vi "UHR-Fleezers Control (host) - 12.8.1.vi"() -> ()   [LabVIEW 2012] (continued)
        n1295 = Path To String(path=w1922) -> (string=w1921:string)
        n1296 = Concatenate Strings(w1921, "\\current.cal" ("string")) -> (w1919:string)
        n1297 = String To Path(string=w1919) -> (path=w1918:path)
        n1298 = Open/Create/Replace File(file path (use dialog)=w1918, operation (0:open)=T33."open", access (0:read/write)=enum16{"read/write", "read-only", "write-only"}."read-only") -> (refnum out=w1926:refnum<file>, error out=w1912:errorcluster)  [unwired: 1 in, 3 out]
        n1299 = Deny Access(4:w1912, 7:w1926) -> (0:w1911:errorcluster, 3:w1917:refnum<file>)  [unwired: 1 out]
        n1300 = Read from Binary File(5:0.0, 8:w1911, 9:T32."big-endian, network order" ("byte order (0:big-endian, network order)"), 10:-1 ("count (1)"), 11:w1917) -> (0:w1910:errorcluster, 2:w1908:dbl[], 3:w1913:refnum<file>)  [unwired: 2 out]
        n1301 = Array To Cluster(array=w1908) -> (cluster=w1907:T35)
        n1302 = Unbundle(w1907) -> ("[0]"=w1901:dbl, "[1]"=w1895:dbl, "[2]"=w1899:dbl, "[3]"=w1893:dbl, "[4]"=w1906:dbl, "[5]"=w1905:dbl)
        n1303 = Close File(refnum=w1913, error in=w1910) -> (error out=→"Read cal error":errorcluster)  [unwired: 1 out]
        n1304 = Multiply(x=w1906, y=w1904) -> (x*y=w1900:dbl)
        n1305 = Multiply(x=w1905, y=w1904) -> (x*y=w1894:dbl)
        n1306 = Bundle By Name(cluster="T1 calibration", "T1 alpha_x (nm/V)"=w1901, "T1 offset_x (mV)"=w1900, "T1 kappa_x (pN/nm)"=w1899) -> (w1898:T6)
        n1307 = Bundle By Name(cluster="T2 calibration", "T2 alpha_x (nm/V)"=w1895, "T2 offset_x (mV)"=w1894, "T2 kappa_x (pN/nm)"=w1893) -> (w1896:T5)
        n1308 = local write "T1 calibration"(w1898) -> ()
        n1309 = local write "T2 calibration"(w1896) -> ()
      }
      event "Abort MCL Scan": Value Change {
        n1310 = event-data() -> ()  [unwired: 7 out]
        n1311 = local write "MCL Scanning"(FALSE ("MCL Scanning")) -> ()
        n1312 = xnode "Read/Write Control"("FPGA VI Reference In"=w1927, "Abort scan (MCL)"="Abort MCL Scan") -> ("error out"=w1930:errorcluster)  [unwired: 1 in, 1 out]
      }
      event "Update Count (MCL)": Value Change {
        n1313 = event-data() -> ()  [unwired: 7 out]
        n1314 = xnode "Read/Write Control"("FPGA VI Reference In"=w1931, "MCL count"="Update Count (MCL)") -> ("error out"=w1933:errorcluster)  [unwired: 1 in, 1 out]
      }
      event "+ phase (MCL)", "- phase (MCL)": Value Change {
        n1315 = event-data() -> ()  [unwired: 7 out]
        n1316 = Or(x="- phase (MCL)", y="+ phase (MCL)") -> (x .or. y?=w1937:bool)
        n1317 = Negate(x="Phase adjust (MCL)") -> (-x=w1943:i16)
        n1318 = Select(t=w1943, s="+ phase (MCL)", f="Phase adjust (MCL)") -> (s? t:f=w1941:i16)
        n1319 = xnode "Read/Write Control"("FPGA VI Reference In"=w1934, "Phase count adjustment (MCL)"=w1941) -> ("FPGA VI Reference Out"=w1938:T24, "error out"=w1939:errorcluster)  [unwired: 1 in]
        n1320 = xnode "Read/Write Control"("FPGA VI Reference In"=w1938, "error in"=w1939, "+ phase (MCL)"=w1937) -> ("error out"=w1936:errorcluster)  [unwired: 1 out]
      }
      event "Abort AOD Scan": Value Change {
        n1321 = event-data() -> ()  [unwired: 7 out]
        n1322 = xnode "Read/Write Control"("FPGA VI Reference In"=w1944, "Abort scan"="Abort AOD Scan") -> ("error out"=w1946:errorcluster)  [unwired: 1 in, 1 out]
      }
      event "Continuous AOD Scanning": Value Change {
        n1323 = event-data() -> ()  [unwired: 7 out]
        n1324 = xnode "Read/Write Control"("FPGA VI Reference In"=w1947, "Cont. Scan"="Continuous AOD Scanning") -> ("error out"=w1949:errorcluster)  [unwired: 1 in, 1 out]
      }
      event "Index": Value Change {
        n1325 = event-data() -> ()  [unwired: 7 out]
        n1326 = call "Create new save file.vi"("Insert"="", "Ext"=".dat" ("string"), "Index In"="Index") -> ("Path Out"=→"Save file name":path, "Index Out"=w1950:dbl)
        "Save index" <- w1950
        n1327 = local write "Index"(w1950) -> ()
      }
      event "AO1", "AO2": Value Change {
        w1964 = 10.0 ("y")
        w1963 = 32767.0 ("y")
        n1328 = event-data() -> ()  [unwired: 7 out]
        n1329 = local read "AO2"() -> (w1962:dbl)
        n1330 = local read "AO1"() -> (w1959:dbl)
        n1331 = Multiply(x=w1959, y=w1963) -> (x*y=w1958:dbl)
        n1332 = Multiply(x=w1962, y=w1963) -> (x*y=w1961:dbl)
        n1333 = Divide(x=w1958, y=w1964) -> (x/y=w1957:dbl)
        n1334 = Divide(x=w1961, y=w1964) -> (x/y=w1960:dbl)
        n1335 = To Word Integer(number=w1957) -> (16bit integer=w1965:i16)
        n1336 = To Word Integer(number=w1960) -> (16bit integer=w1966:i16)
        n1337 = xnode "Read/Write Control"("FPGA VI Reference In"=w1955, "AO1"=w1965, "AO2"=w1966) -> ("error out"=w1956:errorcluster)  [unwired: 1 in, 1 out]
      }
      event "Inject Pump 1": Value Change {
        n1338 = event-data() -> ()  [unwired: 7 out]
        n1339 = local read "Use Harvard pumps\nfor beads (else Chemyx)"() -> (w1968:bool)
        n1340 = case shown="True" w1968 {
          tunnel: "Inject Pump 1" -> [w1972 w2010]
          tunnel: w1967 -> [_ w2011]
          frame False {
            n1341 = local read "Pump write delay (ms)"() -> (w1971:dbl)
            n1342 = local read "Chemyx Syringe Pump Serial Port"() -> (w1970:refnum<visa-resource-name>)
            n1343 = case shown="True" w1972 {
              tunnel: w1971 -> [w1978 w1992]
              tunnel: w1970 -> [w1975 w1991]
              frame False {
                n1344 = flat-sequence {
                  tunnel: w1975 -> [w1979]
                  tunnel: [w1979] -> w1976
                  tunnel: w1978 -> [_]
                  tunnel: [w1982] -> w1977
                  tunnel: w1976 -> [w1982]
                  tunnel: w1977 -> [w1983]
                  tunnel: [w1983] -> w1973
                  tunnel: [w1985] -> w1974
                  tunnel: w1973 -> [w1985]
                  tunnel: w1974 -> [w1987]
                  frame #0 {
                    n1345 = call "Write to pump.vi"("string"="enter pump1", "VISA resource name"=w1979) -> ()  [unwired: 1 out]
                  }
                  frame #1 {
                    n1346 = Wait (ms)(milliseconds to wait="Pump pause delay (ms)") -> ()  [unwired: 1 out]
                  }
                  frame #2 {
                    n1347 = call "Write to pump.vi"("string"="stop", "VISA resource name"=w1983) -> ()  [unwired: 1 out]
                  }
                  frame #3 {
                    n1348 = Wait (ms)(milliseconds to wait=u32 500) -> ()  [unwired: 1 out]
                  }
                  frame #4 {
                    n1349 = call "Write to pump.vi"("string"="stop", "VISA resource name"=w1987) -> ()  [unwired: 1 out]
                  }
                }
              }
              frame True {
                n1350 = flat-sequence {
                  tunnel: w1991 -> [w2001]
                  tunnel: w1992 -> [w1996]
                  tunnel: w1992 -> [w2003]
                  tunnel: w1991 -> [w2004]
                  tunnel: [w2004] -> w1989
                  tunnel: [w2006] -> w1990
                  tunnel: w1989 -> [w2006]
                  tunnel: w1990 -> [w2008]
                  frame #0 {
                    n1351 = local read "All Pump Parameters"() -> (w1995:T7)
                    n1352 = Unbundle By Name(w1995) -> ("Pump 1"=w2002:T36)
                    n1353 = call "Set pump parameters.vi"("Pump write delay (ms)"=w1996, "Volume (uL)"="Ch 1 Inject Volume (uL)", "Rate (uL/h)"="Ch 1 Inject Rate (ul/h)", "Units"=4.0, "Pump #"=1.0, "Pump Parameters In"=w2002, "VISA resource name"=w2001) -> ("Pump Parameters Out"=w1994:T36)  [unwired: 3 in]
                    n1354 = Bundle By Name(cluster=w1995, "Pump 1"=w1994) -> (w1993:T7)
                    n1355 = local write "All Pump Parameters"(w1993) -> ()
                  }
                  frame #1 {
                    n1356 = Wait (ms)(milliseconds to wait=w2003) -> ()  [unwired: 1 out]
                  }
                  frame #2 {
                    n1357 = call "Write to pump.vi"("string"="start", "VISA resource name"=w2004) -> ()  [unwired: 1 out]
                  }
                  frame #3 {
                    n1358 = Wait (ms)(milliseconds to wait=u32 500) -> ()  [unwired: 1 out]
                  }
                  frame #4 {
                    n1359 = call "Write to pump.vi"("string"="start", "VISA resource name"=w2008) -> ()  [unwired: 1 out]
                  }
                }
              }
            }
          }
          frame True {
            n1360 = case shown="False" w2010 {
              tunnel: w2011 -> [w2012 w2022]
              frame False {
                n1361 = flat-sequence {
                  tunnel: w2012 -> [w2014]
                  frame #0 {
                    n1362 = local write "Flushing P1"(FALSE ("Flushing P1")) -> ()
                    n1363 = Concatenate Strings("stop" ("string"), "\r") -> (w2016:string)
                    n1364 = VISA Write(VISA resource name=w2014, write buffer=w2016) -> ()  [unwired: 1 in, 3 out]
                  }
                  frame #1 {
                    n1365 = property on="Clear Volume P1" class="Bool (strict)"("Val(Sgnl)"=TRUE ("Value (Signaling)")) -> ()  [unwired: 2 in, 2 out]
                  }
                }
              }
              frame True {
                n1366 = local read "Normal Flow Rate (ul/h) P1"() -> (w2020:dbl)
                n1367 = Number To Decimal String(number=w2020) -> (decimal integer string=w2026:string)  [unwired: 1 in]
                n1368 = Concatenate Strings("irate  " ("string"), w2026, " u/h" ("string"), "\r") -> (w2024:string)
                n1369 = VISA Write(VISA resource name=w2022, write buffer=w2024) -> (VISA resource name out=w2021:refnum<visa-resource-name>)  [unwired: 1 in, 2 out]
                n1370 = Concatenate Strings("irun" ("string"), "\r") -> (w2028:string)
                n1371 = VISA Write(VISA resource name=w2021, write buffer=w2028) -> ()  [unwired: 1 in, 3 out]
              }
            }
          }
        }
      }
      event "Inject Pump 3": Value Change {
        n1372 = event-data() -> ()  [unwired: 7 out]
        n1373 = local read "Use Harvard pumps\nfor beads (else Chemyx)"() -> (w2031:bool)
        n1374 = case shown="True" w2031 {
          tunnel: "Inject Pump 3" -> [w2035 w2074]
          tunnel: w2030 -> [_ w2073]
          frame False {
            n1375 = local read "Pump write delay (ms)"() -> (w2034:dbl)
            n1376 = case shown="True" w2035 {
              tunnel: w2034 -> [w2041 w2055]
              tunnel: "Chemyx Syringe Pump Serial Port" -> [w2038 w2054]
              frame False {
                n1377 = flat-sequence {
                  tunnel: w2038 -> [w2042]
                  tunnel: [w2042] -> w2039
                  tunnel: w2041 -> [_]
                  tunnel: [w2045] -> w2040
                  tunnel: w2039 -> [w2045]
                  tunnel: w2040 -> [w2046]
                  tunnel: [w2046] -> w2036
                  tunnel: [w2048] -> w2037
                  tunnel: w2036 -> [w2048]
                  tunnel: w2037 -> [w2050]
                  frame #0 {
                    n1378 = call "Write to pump.vi"("string"="enter pump3", "VISA resource name"=w2042) -> ()  [unwired: 1 out]
                  }
                  frame #1 {
                    n1379 = local read "Pump pause delay (ms)"() -> (w2044:u32)
                    n1380 = Wait (ms)(milliseconds to wait=w2044) -> ()  [unwired: 1 out]
                  }
                  frame #2 {
                    n1381 = call "Write to pump.vi"("string"="stop", "VISA resource name"=w2046) -> ()  [unwired: 1 out]
                  }
                  frame #3 {
                    n1382 = Wait (ms)(milliseconds to wait=u32 0) -> ()  [unwired: 1 out]
                  }
                  frame #4 {
                    n1383 = call "Write to pump.vi"("string"="stop", "VISA resource name"=w2050) -> ()  [unwired: 1 out]
                  }
                }
              }
              frame True {
                n1384 = flat-sequence {
                  tunnel: w2054 -> [w2064]
                  tunnel: w2055 -> [w2059]
                  tunnel: w2055 -> [w2066]
                  tunnel: w2054 -> [w2067]
                  tunnel: [w2067] -> w2053
                  tunnel: [w2070] -> w2052
                  tunnel: w2053 -> [w2070]
                  tunnel: w2052 -> [w2071]
                  frame #0 {
                    n1385 = local read "All Pump Parameters"() -> (w2058:T7)
                    n1386 = Unbundle By Name(w2058) -> ("Pump 3"=w2065:T36)
                    n1387 = call "Set pump parameters.vi"("Pump write delay (ms)"=w2059, "Volume (uL)"="Ch 3 Inject Volume (uL)", "Rate (uL/h)"="Ch 3 Inject Rate (ul/h)", "Units"=4.0, "Pump #"=3.0, "Pump Parameters In"=w2065, "VISA resource name"=w2064) -> ("Pump Parameters Out"=w2057:T36)  [unwired: 3 in]
                    n1388 = Bundle By Name(cluster=w2058, "Pump 3"=w2057) -> (w2056:T7)
                    n1389 = local write "All Pump Parameters"(w2056) -> ()
                  }
                  frame #1 {
                    n1390 = Wait (ms)(milliseconds to wait=w2066) -> ()  [unwired: 1 out]
                  }
                  frame #2 {
                    n1391 = call "Write to pump.vi"("string"="start", "VISA resource name"=w2067) -> ()  [unwired: 1 out]
                  }
                  frame #3 {
                    n1392 = Wait (ms)(milliseconds to wait=u32 500) -> ()  [unwired: 1 out]
                  }
                  frame #4 {
                    n1393 = call "Write to pump.vi"("string"="start", "VISA resource name"=w2071) -> ()  [unwired: 1 out]
                  }
                }
              }
            }
          }
          frame True {
            n1394 = case shown="False" w2074 {
              tunnel: w2073 -> [w2075 w2082]
              frame False {
                n1395 = flat-sequence {
                  tunnel: w2075 -> [w2077]
                  frame #0 {
                    n1396 = local write "Flushing P3"(FALSE ("Flushing P3")) -> ()
                    n1397 = Concatenate Strings("stop" ("string"), "\r") -> (w2079:string)
                    n1398 = VISA Write(VISA resource name=w2077, write buffer=w2079) -> ()  [unwired: 1 in, 3 out]
                  }
                  frame #1 {
                    n1399 = property on="Clear Volume P3" class="Bool (strict)"("Val(Sgnl)"=TRUE ("Value (Signaling)")) -> ()  [unwired: 2 in, 2 out]
                  }
                }
              }
              frame True {
                n1400 = local read "Normal Flow Rate (ul/h) P3"() -> (w2083:dbl)
                n1401 = Number To Decimal String(number=w2083) -> (decimal integer string=w2089:string)  [unwired: 1 in]
                n1402 = Concatenate Strings("irate  " ("string"), w2089, " u/h" ("string"), "\r") -> (w2087:string)
                n1403 = VISA Write(VISA resource name=w2082, write buffer=w2087) -> (VISA resource name out=w2085:refnum<visa-resource-name>)  [unwired: 1 in, 2 out]
                n1404 = Concatenate Strings("irun" ("string"), "\r") -> (w2091:string)
                n1405 = VISA Write(VISA resource name=w2085, write buffer=w2091) -> ()  [unwired: 1 in, 3 out]
              }
            }
          }
        }
      }
      event "Inject Pump 2": Value Change {
        n1406 = event-data() -> ()  [unwired: 7 out]
        n1407 = local read "Pump write delay (ms)"() -> (w2095:dbl)
        n1408 = flat-sequence {
          tunnel: w2093 -> [w2108]
          tunnel: w2095 -> [w2104]
          tunnel: "Inject Pump 2" -> [_]
          tunnel: w2095 -> [w2110]
          tunnel: w2093 -> [w2111]
          frame #0 {
            n1409 = local read "All Pump Parameters"() -> (w2103:T7)
            n1410 = Multiply(x=60.0, y="Flush Center Ch Rate (ul/m)") -> (x*y=w2100:dbl)
            n1411 = Unbundle By Name(w2103) -> ("Pump 2"=w2109:T36)
            n1412 = call "Set pump parameters.vi"("Pump write delay (ms)"=w2104, "Volume (uL)"="Flush Center Ch Volume (uL)", "Rate (uL/h)"=w2100, "Units"=3.0, "Pump #"=2.0, "Pump Parameters In"=w2109, "VISA resource name"=w2108) -> ("Pump Parameters Out"=w2102:T36)  [unwired: 3 in]
            n1413 = Bundle By Name(cluster=w2103, "Pump 2"=w2102) -> (w2101:T7)
            n1414 = local write "All Pump Parameters"(w2101) -> ()
            n1415 = Add(x="Flush Center Ch Volume (uL)", y="Total Volume\nFlushed (uL)") -> (x+y=w2097:dbl)
            n1416 = local write "Total Volume\nFlushed (uL)"(w2097) -> ()
          }
          frame #1 {
            n1417 = Wait (ms)(milliseconds to wait=w2110) -> ()  [unwired: 1 out]
          }
          frame #2 {
            n1418 = call "Write to pump.vi"("string"="start", "VISA resource name"=w2111) -> ()  [unwired: 1 out]
          }
        }
        n1419 = local read "Chemyx Syringe Pump Serial Port"() -> (w2093:refnum<visa-resource-name>)
      }
      event "Sample Channel\nFlow": Value Change {
        n1420 = event-data() -> ()  [unwired: 7 out]
        n1421 = Select(t="irun" ("string"), s="Sample Channel\nFlow", f="stop" ("string")) -> (s? t:f=w2115:string)
        n1422 = Concatenate Strings(w2115, "\r") -> (w2118:string)
        n1423 = VISA Write(VISA resource name=w2113, write buffer=w2118) -> ()  [unwired: 1 in, 3 out]
      }
      event "Start Flow": Value Change {
        n1424 = event-data() -> ()  [unwired: 7 out]
        n1425 = local write "Sample Channel\nFlow"(TRUE ("Sample Channel\nFlow")) -> ()
        n1426 = local write "Start Flow"(FALSE ("Start Flow")) -> ()
        n1427 = Concatenate Strings("irun" ("string"), "\r") -> (w2124:string)
        n1428 = VISA Write(VISA resource name=w2120, write buffer=w2124) -> ()  [unwired: 1 in, 3 out]
      }
      event "Stop Flow": Value Change {
        w2126 = FALSE ("Stop Flow")
        n1429 = event-data() -> ()  [unwired: 7 out]
        n1430 = local write "Stop Flow"(w2126) -> ()
        n1431 = local write "Sample Channel\nFlow"(w2126) -> ()
        n1432 = Concatenate Strings("stop" ("string"), "\r") -> (w2129:string)
        n1433 = VISA Write(VISA resource name=w2127, write buffer=w2129) -> ()  [unwired: 1 in, 3 out]
      }
      event "Flow rate (uL/h)": Value Change {
        n1434 = event-data() -> ()  [unwired: 7 out]
        n1435 = Number To Decimal String(number="Flow rate (uL/h)") -> (decimal integer string=w2136:string)  [unwired: 1 in]
        n1436 = Concatenate Strings("irate  " ("string"), w2136, " u/h" ("string"), "\r") -> (w2135:string)
        n1437 = VISA Write(VISA resource name=w2132, write buffer=w2135) -> ()  [unwired: 1 in, 3 out]
      }
      event "Flush Sample": Value Change {
        n1438 = event-data() -> ()  [unwired: 7 out]
        n1439 = flat-sequence {
          tunnel: w2141 -> [w2169]
          tunnel: [w2149] -> w2140
          tunnel: [w2143] -> w2138
          tunnel: w2140 -> [w2173]
          tunnel: [w2173] -> w2139
          tunnel: w2138 -> [w2172]
          tunnel: w2139 -> [w2178]
          frame #0 {
            # "set paramaters (rate, volume) for flush, clear volume"
            n1440 = Number To Decimal String(number="Flush rate (uL/m)") -> (decimal integer string=w2165:string)  [unwired: 1 in]
            n1441 = Concatenate Strings("irate  " ("string"), w2165, " u/m" ("string"), "\r") -> (w2167:string)
            n1442 = VISA Write(VISA resource name=w2169, write buffer=w2167) -> (VISA resource name out=w2163:refnum<visa-resource-name>)  [unwired: 1 in, 2 out]
            n1443 = Reciprocal(x="Flush rate (uL/m)") -> (1/x=w2146:dbl)
            n1444 = Number To Decimal String(number="Volume (uL)") -> (decimal integer string=w2154:string)  [unwired: 1 in]
            n1445 = Multiply(x="Volume (uL)", y=w2146) -> (x*y=w2145:dbl)
            n1446 = Concatenate Strings("tvolume  " ("string"), w2154, " u" ("string"), "\r") -> (w2152:string)
            n1447 = Multiply(x=w2145, y=60000.0) -> (x*y=w2143:dbl)
            n1448 = VISA Write(VISA resource name=w2163, write buffer=w2152) -> (VISA resource name out=w2151:refnum<visa-resource-name>)  [unwired: 1 in, 2 out]
            n1449 = Concatenate Strings("cvolume" ("string"), "\r") -> (w2150:string)
            n1450 = VISA Write(VISA resource name=w2151, write buffer=w2150) -> (VISA resource name out=w2161:refnum<visa-resource-name>)  [unwired: 1 in, 2 out]
            n1451 = Concatenate Strings("irun" ("string"), "\r") -> (w2159:string)
            n1452 = VISA Write(VISA resource name=w2161, write buffer=w2159) -> (VISA resource name out=w2149:refnum<visa-resource-name>)  [unwired: 1 in, 2 out]
          }
          frame #1 {
            # "Have to wait until\nflow is done to reset\nrate"
            n1453 = Add(x=w2172, y=100.0) -> (x+y=w2171:dbl)
            n1454 = Wait (ms)(milliseconds to wait=w2171) -> ()  [unwired: 1 out]
          }
          frame #2 {
            # "reset flow rate to usual flow rate"
            n1455 = local read "Flow rate (uL/h)"() -> (w2184:dbl)
            n1456 = Number To Decimal String(number=w2184) -> (decimal integer string=w2182:string)  [unwired: 1 in]
            n1457 = Concatenate Strings("irate  " ("string"), w2182, " u/h" ("string"), "\r") -> (w2180:string)
            n1458 = VISA Write(VISA resource name=w2178, write buffer=w2180) -> (VISA resource name out=w2174:refnum<visa-resource-name>)  [unwired: 1 in, 2 out]
            n1459 = Concatenate Strings("cvolume" ("string"), "\r") -> (w2175:string)
            n1460 = VISA Write(VISA resource name=w2174, write buffer=w2175) -> ()  [unwired: 1 in, 3 out]
          }
        }
      }
      event "Flush Pump 3": Value Change {
        n1461 = event-data() -> ()  [unwired: 7 out]
        n1462 = flat-sequence {
          tunnel: w2185 -> [w2188]
          frame #0 {
            # "set paramaters (rate, volume) for flush, clear volume"
            n1463 = Number To Decimal String(number="Flush rate (uL/m) P3") -> (decimal integer string=w2210:string)  [unwired: 1 in]
            n1464 = local write "Inject Pump 3"(TRUE ("Inject Pump 3")) -> ()
            n1465 = Concatenate Strings("irate  " ("string"), w2210, " u/m" ("string"), "\r") -> (w2212:string)
            n1466 = VISA Write(VISA resource name=w2188, write buffer=w2212) -> (VISA resource name out=w2208:refnum<visa-resource-name>)  [unwired: 1 in, 2 out]
            n1467 = Reciprocal(x="Flush rate (uL/m) P3") -> (1/x=w2192:dbl)
            n1468 = Number To Decimal String(number="Volume (uL) P3") -> (decimal integer string=w2199:string)  [unwired: 1 in]
            n1469 = Multiply(x="Volume (uL) P3", y=w2192) -> (x*y=w2191:dbl)
            n1470 = Concatenate Strings("tvolume  " ("string"), w2199, " u" ("string"), "\r") -> (w2197:string)
            n1471 = Multiply(x=w2191, y=60.0) -> (x*y=→"HP3 Flush Time (s)":dbl)
            n1472 = VISA Write(VISA resource name=w2208, write buffer=w2197) -> (VISA resource name out=w2196:refnum<visa-resource-name>)  [unwired: 1 in, 2 out]
            n1473 = Concatenate Strings("cvolume" ("string"), "\r") -> (w2195:string)
            n1474 = VISA Write(VISA resource name=w2196, write buffer=w2195) -> (VISA resource name out=w2206:refnum<visa-resource-name>)  [unwired: 1 in, 2 out]
            n1475 = Concatenate Strings("irun" ("string"), "\r") -> (w2204:string)
            n1476 = VISA Write(VISA resource name=w2206, write buffer=w2204) -> ()  [unwired: 1 in, 3 out]
          }
          frame #1 {
            "Flushing P3" <- TRUE ("Flushing P3")
          }
        }
      }
      event "Flush Pump 1": Value Change {
        n1477 = event-data() -> ()  [unwired: 7 out]
        n1478 = flat-sequence {
          tunnel: [w2226] -> w2216
          tunnel: w2215 -> [w2219]
          tunnel: w2216 -> [_]
          frame #0 {
            # "set paramaters (rate, volume) for flush, clear volume"
            n1479 = local write "Inject Pump 1"(TRUE ("Inject Pump 1")) -> ()
            n1480 = Number To Decimal String(number="Flush rate (uL/m) P1") -> (decimal integer string=w2242:string)  [unwired: 1 in]
            n1481 = Concatenate Strings("irate  " ("string"), w2242, " u/m" ("string"), "\r") -> (w2244:string)
            n1482 = VISA Write(VISA resource name=w2219, write buffer=w2244) -> (VISA resource name out=w2240:refnum<visa-resource-name>)  [unwired: 1 in, 2 out]
            n1483 = Reciprocal(x="Flush rate (uL/m) P1") -> (1/x=w2223:dbl)
            n1484 = Number To Decimal String(number="Volume (uL) P1") -> (decimal integer string=w2231:string)  [unwired: 1 in]
            n1485 = Multiply(x="Volume (uL) P1", y=w2223) -> (x*y=w2222:dbl)
            n1486 = Concatenate Strings("tvolume  " ("string"), w2231, " u" ("string"), "\r") -> (w2229:string)
            n1487 = Multiply(x=w2222, y=60.0) -> (x*y=→"HP1 Flush Time (s)":dbl)
            n1488 = VISA Write(VISA resource name=w2240, write buffer=w2229) -> (VISA resource name out=w2228:refnum<visa-resource-name>)  [unwired: 1 in, 2 out]
            n1489 = Concatenate Strings("cvolume" ("string"), "\r") -> (w2227:string)
            n1490 = VISA Write(VISA resource name=w2228, write buffer=w2227) -> (VISA resource name out=w2238:refnum<visa-resource-name>)  [unwired: 1 in, 2 out]
            n1491 = Concatenate Strings("irun" ("string"), "\r") -> (w2236:string)
            n1492 = VISA Write(VISA resource name=w2238, write buffer=w2236) -> (VISA resource name out=w2226:refnum<visa-resource-name>)  [unwired: 1 in, 2 out]
          }
          frame #1 {
            "Flushing P1" <- TRUE ("Flushing P3")
          }
        }
      }
      event "Clear Volume": Value Change {
        n1493 = event-data() -> ()  [unwired: 7 out]
        n1494 = Concatenate Strings("cvolume" ("string"), "\r") -> (w2248:string)
        n1495 = VISA Write(VISA resource name=w2247, write buffer=w2248) -> ()  [unwired: 1 in, 3 out]
      }
      event "Clear Volume P3": Value Change {
        n1496 = event-data() -> ()  [unwired: 7 out]
        n1497 = Concatenate Strings("cvolume" ("string"), "\r") -> (w2254:string)
        n1498 = VISA Write(VISA resource name=w2253, write buffer=w2254) -> ()  [unwired: 1 in, 3 out]
        n1499 = local write "Clear Volume P3"(FALSE ("Clear Volume P3")) -> ()
      }
      event "Clear Volume P1": Value Change {
        n1500 = event-data() -> ()  [unwired: 7 out]
        n1501 = Concatenate Strings("cvolume" ("string"), "\r") -> (w2259:string)
        n1502 = local write "Clear Volume P1"(FALSE ("Clear Volume P1")) -> ()
        n1503 = VISA Write(VISA resource name=w2258, write buffer=w2259) -> ()  [unwired: 1 in, 3 out]
      }
      event "Display On P3": Value Change {
        n1504 = event-data() -> ()  [unwired: 7 out]
        n1505 = Select(t="dim 100", s="Display On P3", f="dim 0") -> (s? t:f=w2265:string)
        n1506 = Concatenate Strings(w2265, "\r") -> (w2267:string)
        n1507 = VISA Write(VISA resource name=w2262, write buffer=w2267) -> ()  [unwired: 1 in, 3 out]
      }
      event "Display On P1": Value Change {
        n1508 = event-data() -> ()  [unwired: 7 out]
        n1509 = Select(t="dim 100", s="Display On P1", f="dim 0") -> (s? t:f=w2272:string)
        n1510 = Concatenate Strings(w2272, "\r") -> (w2274:string)
        n1511 = VISA Write(VISA resource name=w2269, write buffer=w2274) -> ()  [unwired: 1 in, 3 out]
      }
      event "Retract Pump 3": Value Change {
        n1512 = event-data() -> ()  [unwired: 7 out]
        n1513 = local write "Retract Pump 3"(FALSE ("Retract Pump 3")) -> ()
        n1514 = case shown="True" "Retract Pump 3" {
          tunnel: w2276 -> [_ w2279]
          frame False {
          }
          frame True {
            n1515 = Number To Decimal String(number="Retract Rate (uL/m)") -> (decimal integer string=w2297:string)  [unwired: 1 in]
            n1516 = Concatenate Strings("wrate  " ("string"), w2297, " u/m" ("string"), "\r") -> (w2299:string)
            n1517 = VISA Write(VISA resource name=w2279, write buffer=w2299) -> (VISA resource name out=w2290:refnum<visa-resource-name>)  [unwired: 1 in, 2 out]
            n1518 = Number To Decimal String(number="Retract Vol 3 (uL)") -> (decimal integer string=w2292:string)  [unwired: 1 in]
            n1519 = Concatenate Strings("tvolume  " ("string"), w2292, " u" ("string"), "\r") -> (w2289:string)
            n1520 = VISA Write(VISA resource name=w2290, write buffer=w2289) -> (VISA resource name out=w2285:refnum<visa-resource-name>)  [unwired: 1 in, 2 out]
            n1521 = Concatenate Strings("cvolume" ("string"), "\r") -> (w2286:string)
            n1522 = VISA Write(VISA resource name=w2285, write buffer=w2286) -> (VISA resource name out=w2280:refnum<visa-resource-name>)  [unwired: 1 in, 2 out]
            n1523 = Concatenate Strings("wrun" ("string"), "\r") -> (w2281:string)
            n1524 = VISA Write(VISA resource name=w2280, write buffer=w2281) -> ()  [unwired: 1 in, 3 out]
          }
        }
      }
      event "Retract Pump 1": Value Change {
        n1525 = event-data() -> ()  [unwired: 7 out]
        n1526 = local write "Retract Pump 1"(FALSE ("Retract Pump 1")) -> ()
        n1527 = case shown="True" "Retract Pump 1" {
          tunnel: w2301 -> [_ w2306]
          frame False {
          }
          frame True {
            n1528 = local read "Retract Rate (uL/m)"() -> (w2304:dbl)
            n1529 = Number To Decimal String(number=w2304) -> (decimal integer string=w2322:string)  [unwired: 1 in]
            n1530 = Concatenate Strings("wrate  " ("string"), w2322, " u/m" ("string"), "\r") -> (w2324:string)
            n1531 = VISA Write(VISA resource name=w2306, write buffer=w2324) -> (VISA resource name out=w2316:refnum<visa-resource-name>)  [unwired: 1 in, 2 out]
            n1532 = Number To Decimal String(number="Retract Vol 1 (uL)") -> (decimal integer string=w2318:string)  [unwired: 1 in]
            n1533 = Concatenate Strings("tvolume  " ("string"), w2318, " u" ("string"), "\r") -> (w2315:string)
            n1534 = VISA Write(VISA resource name=w2316, write buffer=w2315) -> (VISA resource name out=w2312:refnum<visa-resource-name>)  [unwired: 1 in, 2 out]
            n1535 = Concatenate Strings("cvolume" ("string"), "\r") -> (w2313:string)
            n1536 = VISA Write(VISA resource name=w2312, write buffer=w2313) -> (VISA resource name out=w2307:refnum<visa-resource-name>)  [unwired: 1 in, 2 out]
            n1537 = Concatenate Strings("wrun" ("string"), "\r") -> (w2308:string)
            n1538 = VISA Write(VISA resource name=w2307, write buffer=w2308) -> ()  [unwired: 1 in, 3 out]
          }
        }
      }
      event "Flip Green Filter": Value Change {
        n1539 = event-data() -> ()  [unwired: 7 out]
        n1540 = Not(x="Flip Green Filter") -> (.not. x?=w2327:bool)
        n1541 = local write "Flip Green Filter"(w2327) -> ()
        n1542 = flat-sequence {
          tunnel: [w2336] -> w2332
          tunnel: [w2335] -> w2331
          tunnel: w2326 -> [w2334]
          tunnel: [w2339] -> w2330
          tunnel: w2332 -> [w2339]
          tunnel: [w2338] -> w2329
          tunnel: w2331 -> [w2338]
          tunnel: w2330 -> [w2343]
          tunnel: w2329 -> [w2342]
          tunnel: [w2341] -> w2333
          frame #0 {
            n1543 = xnode "Read/Write Control"("FPGA VI Reference In"=w2334, "Green Filter Flipper"=TRUE) -> ("FPGA VI Reference Out"=w2336:T24, "error out"=w2335:errorcluster)  [unwired: 1 in]
          }
          frame #1 {
            n1544 = Wait (ms)(milliseconds to wait=u32 100) -> ()  [unwired: 1 out]
          }
          frame #2 {
            n1545 = xnode "Read/Write Control"("FPGA VI Reference In"=w2343, "error in"=w2342, "Green Filter Flipper"=FALSE) -> ("error out"=w2341:errorcluster)  [unwired: 1 out]
          }
        }
      }
      event "Pump 1 contents", "Pump 3 contents": Value Change {
        n1546 = event-data() -> ()  [unwired: 7 out]
        n1547 = local read "Pump 1 contents"() -> (→"Pump 1 cont disp":string)
        n1548 = local read "Pump 3 contents"() -> (→"Pump 3 cont disp":string)
      }
      event "Reset Trap Pos. FB": Value Change {
        n1549 = event-data() -> ()  [unwired: 7 out]
        n1550 = xnode "Read/Write Control"("FPGA VI Reference In"=w2347, "Trap Pos. FB Reset"="Reset Trap Pos. FB") -> ()  [unwired: 1 in, 2 out]
      }
      event "Rem fb disp offset": Value Change {
        n1551 = event-data() -> ()  [unwired: 7 out]
        n1552 = local write "Rem fb disp offset"(FALSE ("Rem fb disp offset")) -> ()
        n1553 = local read "Mean T1 Position (nm)"() -> (w2350:dbl)
        n1554 = local read "FB Trap Pos Offset"() -> (w2351:dbl)
        n1555 = Subtract(x=w2351, y=w2350) -> (x-y=w2349:dbl)
        n1556 = local write "FB Trap Pos Offset"(w2349) -> ()
      }
      event "Threshold (nm)": Value Change {
        n1557 = event-data() -> ()  [unwired: 7 out]
        n1558 = flat-sequence {
          tunnel: [w2356] -> w2354
          tunnel: w2353 -> [w2355]
          tunnel: w2354 -> [w2367]
          frame #0 {
            n1559 = xnode "Read/Write Control"("FPGA VI Reference In"=w2355) -> ("FPGA VI Reference Out"=w2359:T24, "error out"=w2358:errorcluster, "FPGA TTrig Thresh"=w2360:i64)  [unwired: 1 in]
            n1560 = local read "Threshold stored (nm)"() -> (w2366:dbl)
            n1561 = local read "Threshold (nm)"() -> (w2356:dbl)
            n1562 = local read "AOM X Cal (nm/MHz)"() -> (w2364:dbl)
            n1563 = Subtract(x=w2356, y=w2366) -> (x-y=w2365:dbl)
            n1564 = Divide(x=w2365, y=w2364) -> (x/y=w2362:dbl)
            n1565 = call "IR AOM freq to word.vi"("Frequency In (MHz)"=w2362) -> ("Frequency Word Out (double)"=w2363:dbl)
            n1566 = To Quad Integer(1:w2363) -> (0:w2361:i64)
            n1567 = Add(x=w2360, y=w2361) -> (x+y=w2357:i64)
            n1568 = xnode "Read/Write Control"("FPGA VI Reference In"=w2359, "error in"=w2358, "FPGA TTrig Thresh"=w2357) -> ()  [unwired: 2 out]
          }
          frame #1 {
            "Threshold stored (nm)" <- w2367
          }
        }
      }
      event "FB Trig Integrate": Value Change {
        n1569 = event-data() -> ()  [unwired: 7 out]
        n1570 = local read "FB Trig Integrate"() -> (w2370:u32)
        n1571 = xnode "Read/Write Control"("FPGA VI Reference In"=w2368, "FB Trig Integrate"=w2370) -> ("error out"=w2369:errorcluster)  [unwired: 1 in, 1 out]
      }
      event "11": Value Change {
        n1572 = event-data() -> ()  [unwired: 7 out]
        n1573 = local read "11"() -> (w2371:bool)
        n1574 = case shown="True" w2371 {
          frame False {
          }
          frame True {
            n1575 = local read "Messages"() -> (w2373:string)
            n1576 = call "Update messages.vi"("Message to add"="You kicked it up to 11!", "Old message string"=w2373) -> ("New message string"=w2374:string)
            n1577 = call <vilib>:"Beep.vi"() -> ()  [unwired: 12 in]
            n1578 = local write "Messages"(w2374) -> ()
          }
        }
      }
      event "Trap Pos. FB ON": Value Change {
        n1579 = event-data() -> ()  [unwired: 7 out]
        n1580 = xnode "Read/Write Control"("FPGA VI Reference In"=w2375, "Force feedback"="Trap Pos. FB ON") -> ()  [unwired: 1 in, 2 out]
      }
      event "Remove Action Offset": Value Change {
        n1581 = event-data() -> ()  [unwired: 7 out]
        n1582 = local write "Remove Action Offset"(FALSE ("Remove Action Offset")) -> ()
        n1583 = local read "Trap Pos. FB Mult Factor"() -> (w2382:i64)
        n1584 = local read "Trap Pos FB Action"() -> (w2380:i64)
        n1585 = local read "Trap Pos. FB Offset Factor"() -> (w2378:i64)
        n1586 = Multiply(x=w2382, y=w2380) -> (x*y=w2381:i64)
        n1587 = Add(x=w2381, y=w2378) -> (x+y=w2379:i64)
        n1588 = local write "Trap Pos. FB Offset Factor"(w2379) -> ()
        n1589 = xnode "Read/Write Control"("FPGA VI Reference In"=w2377, "Trap Pos. FB Offset Factor"=w2379) -> ()  [unwired: 1 in, 2 out]
      }
      event "Remove Unwinding Offset": Value Change {
        n1590 = event-data() -> ()  [unwired: 7 out]
        n1591 = local write "Remove Unwinding Offset"(FALSE ("Remove Action Offset")) -> ()
        n1592 = local read "Trap Pos. FB Mult Factor"() -> (w2396:i64)
        n1593 = local read "Trap Pos FB Action"() -> (w2394:i64)
        n1594 = local read "Trap Pos. FB Offset Factor"() -> (w2393:i64)
        n1595 = Multiply(x=w2396, y=w2394) -> (x*y=w2395:i64)
        n1596 = local read "Trap Pos. FB Mult Factor"() -> (w2392:i64)
        n1597 = Add(x=w2395, y=w2393) -> (x+y=w2386:i64)
        n1598 = Multiply(x=32768, y="factor") -> (x*y=w2389:dbl)
        n1599 = Multiply(x=w2389, y=w2392) -> (x*y=w2391:dbl)
        n1600 = Subtract(x=w2386, y=w2391) -> (x-y=w2390:dbl)
        n1601 = To Quad Integer(1:w2390) -> (0:w2385:i64)
        n1602 = xnode "Read/Write Control"("FPGA VI Reference In"=w2384, "Trap Pos. FB Offset Factor"=w2385) -> ()  [unwired: 1 in, 2 out]
        n1603 = local write "Trap Pos. FB Offset Factor"(w2385) -> ()
      }
      event "Trap Pos. FB Range", "Trap Pos. FB Gains", "Trap Pos. FB Mult Factor", "Trap Pos. FB Offset Factor", "Trap Pos FB Negate Action", "Trap Pos FB Monitor\nT1 or T2", "Differential FB?", "Negate Diff?": Value Change {
        n1604 = event-data() -> ()  [unwired: 7 out]
        n1605 = Unbundle By Name("Trap Pos. FB Gains") -> ("proportional gain (Kc)"=w2401:fxp<+/-,16,8>, "integral gain (Kc*Ts/Ti)"=w2400:fxp<+/-,16,8>, "derivative gain (Kc*Td/Ts)"=w2399:fxp<+/-,16,8>)
        n1606 = local read "Negate Diff?"() -> (w2406:bool)
        n1607 = Unbundle By Name("Trap Pos. FB Range") -> ("output high"=w2404:fxp<+/-,16,1>, "output low"=w2403:fxp<+/-,16,1>)
        n1608 = xnode "Read/Write Control"("FPGA VI Reference In"=w2398, "FB2 output high"=w2404, "FB2 output low"=w2403, "P2"=w2401, "I2"=w2400, "D2"=w2399, "Trap Pos. FB Mult Factor"="Trap Pos. FB Mult Factor", "Trap Pos. FB Offset Factor"="Trap Pos. FB Offset Factor", "Trap Pos FB Negate Action"="Trap Pos FB Negate Action", "Trap Pos FB Monitor T1 or T2"="Trap Pos FB Monitor\nT1 or T2", "AI1 X Scale"="Trap Pos. AI1 X Pre-scale", "Negate Diff?"=w2406, "Diff FB Measurement?"="Differential FB?") -> ()  [unwired: 1 in, 2 out]
      }
      event "Trap Pos FB SP", "Trap Pos FB SP 2", "Use SP 2": Value Change {
        n1609 = event-data() -> ()  [unwired: 7 out]
        n1610 = Select(t="Trap Pos FB SP 2", s="Use SP 2", f="Trap Pos FB SP") -> (s? t:f=w2414:fxp<+/-,16,1>)
        n1611 = xnode "Read/Write Control"("FPGA VI Reference In"=w2413, "Trap Pos. FB SP"=w2414) -> ()  [unwired: 1 in, 2 out]
      }
      event "Offset SP2 from SP1": Value Change {
        n1612 = event-data() -> ()  [unwired: 7 out]
        n1613 = local read "Trap Pos FB SP"() -> (w2420:fxp<+/-,16,1>)
        n1614 = Add(x=w2420, y="SP2 Offset") -> (x+y=w2418:fxp<+/-,16,1>)
        n1615 = property on="Trap Pos FB SP 2" class="DigNum (strict)"("Val(Sgnl)"=w2418) -> ()  [unwired: 2 in, 2 out]
        n1616 = local write "Offset SP2 from SP1"(FALSE ("Offset SP2 from SP1")) -> ()
      }
      event "Set Reading to\nSetpoint": Value Change {
        # "This is the actual PID input signal"
        n1617 = event-data() -> ()  [unwired: 7 out]
        n1618 = local write "Set Reading to\nSetpoint"(FALSE ("Set SP to Reading")) -> ()
        n1619 = xnode "Read/Write Control"("FPGA VI Reference In"=w2422) -> ("FPGA VI Reference Out"=w2425:T24, "error out"=w2424:errorcluster, "Trap Pos FB Int-Norm Signal"=w2423:fxp<+/-,16,1>)  [unwired: 1 in]
        n1620 = local read "Differential FB?"() -> (w2426:bool)
        n1621 = case shown="False" w2426 {
          tunnel: [w2431 w2438] -> w2428
          tunnel: w2423 -> [w2429 w2438]
          frame False {
            n1622 = local read "Trap Pos FB Monitor\nT1 or T2"() -> (w2434:bool)
            n1623 = local read "Trap X AI1 (DMA)"() -> (w2437:T15)
            n1624 = Unbundle By Name(w2437) -> ("Set 1"=w2436:fxp<+/-,16,1>, "Set 2"=w2435:fxp<+/-,16,1>)
            n1625 = Select(t=w2436, s=w2434, f=w2435) -> (s? t:f=w2433:fxp<+/-,16,1>)
            n1626 = Not(x="Set SP Using...") -> (.not. x?=w2430:bool)
            n1627 = Select(t=w2429, s=w2430, f=w2433) -> (s? t:f=w2431:fxp<+/-,16,1>)
          }
          frame True {
          }
        }
        n1628 = xnode "Read/Write Control"("FPGA VI Reference In"=w2425, "error in"=w2424, "Trap Pos. FB SP"=w2428) -> ()  [unwired: 2 out]
        n1629 = local write "Trap Pos FB SP"(w2428) -> ()
      }
      event "Trap Pos. FB Out Scale 2^n": Value Change {
        n1630 = event-data() -> ()  [unwired: 7 out]
        n1631 = Scale By Power Of 2(n="Trap Pos. FB Out Scale 2^n", x=ext 1.0) -> (x*2^n=w2439:ext)
        n1632 = property on="Trap Pos. FB Mult Factor" class="DigNum (strict)"("Val(Sgnl)"=w2439) -> ()  [unwired: 2 in, 2 out]
      }
      event "Trap Pos FB Int Count": Value Change {
        n1633 = event-data() -> ()  [unwired: 7 out]
        n1634 = xnode "Read/Write Control"("FPGA VI Reference In"=w2442, "Trap Pos FB Int Count"="Trap Pos FB Int Count") -> ()  [unwired: 1 in, 2 out]
      }
      event "Trap pos": Value Change {
        n1635 = event-data() -> ()  [unwired: 7 out]
        n1636 = case shown="True" "Trap pos" {
          frame False {
            n1637 = property on="Trap Delta Graph" class="WFGraph (strict)"("Visible"=TRUE) -> ()  [unwired: 2 in, 2 out]
            n1638 = property on="Saved trap pos" class="WFGraph (strict)"("Visible"=FALSE) -> ()  [unwired: 2 in, 2 out]
          }
          frame True {
            n1639 = property on="Saved trap pos" class="WFGraph (strict)"("Visible"=TRUE) -> ()  [unwired: 2 in, 2 out]
            n1640 = property on="Trap Delta Graph" class="WFGraph (strict)"("Visible"=FALSE) -> ()  [unwired: 2 in, 2 out]
          }
        }
      }
      event "Calibration": Value Change {
        n1641 = event-data() -> ()  [unwired: 7 out]
        n1642 = local read "X or Y?"() -> (w2465:bool)
        n1643 = local read "Calibration"() -> (w2462:u16)
        n1644 = Select(t="X" ("Label.Text"), s=w2465, f="Y" ("Label.Text")) -> (s? t:f=w2459:string)
        n1645 = case shown="0, Default" w2462 {
          tunnel: ["Position (V)" ("Label.Text") "Position (nm)" ("Label.Text") "Force (pN)" ("Label.Text")] -> w2456
          tunnel: [" (V)" ("Label.Text") " (nm)" ("Label.Text") " (pN)" ("Label.Text")] -> w2453
          frame 0, Default {
          }
          frame 1 {
          }
          frame 2 {
          }
        }
        n1646 = Concatenate Strings("T1 " ("Label.Text"), w2459) -> (w2455:string)
        n1647 = Concatenate Strings("T2 " ("Label.Text"), w2459) -> (w2454:string)
        n1648 = property on="Force" class="WFChart (strict)"("YScale.NameLbl.Text"=w2456) -> ()  [unwired: 2 in, 2 out]
        n1649 = Concatenate Strings("Mean" ("Label.Text"), w2453) -> (w2452:string)
        n1650 = Concatenate Strings(w2455, w2453) -> (w2451:string)
        n1651 = Concatenate Strings(w2454, w2453) -> (w2450:string)
        n1652 = Concatenate Strings("Difference" ("Label.Text"), w2453) -> (w2449:string)
        n1653 = property on="Mean" class="DigNum (strict)"("Caption.Text"=w2452) -> ()  [unwired: 2 in, 2 out]
        n1654 = property on="T1 X" class="DigNum (strict)"("Caption.Text"=w2451) -> ()  [unwired: 2 in, 2 out]
        n1655 = property on="T2 X" class="DigNum (strict)"("Caption.Text"=w2450) -> ()  [unwired: 2 in, 2 out]
        n1656 = property on="Difference" class="DigNum (strict)"("Caption.Text"=w2449) -> ()  [unwired: 2 in, 2 out]
      }
    }
    "error out 2" <- w1305
    n1657 = node-c288() -> ()  [unwired: 2 out]
  }
  n1658 = timed-loop "Rough control of MCL mirror stage (debugging)" {
    tunnel: [w2474] -> w88
    timing: w34 -> [_]
    timing-out: [_] -> w33
    tunnel: w17 -> [w2472]
    stop <- w2474 stop-if-true
    n1659 = node-c288() -> ()  [unwired: 2 out]
    n1660 = case shown="2" "MCL Mode" {
      tunnel: w2472 -> [_ w2477 w2524]
      frame 0, Default {
      }
      frame 1 {
        n1661 = node-c288() -> (w2479:T27)  [unwired: 4 out]
        n1662 = timed-loop "Oscillate MCL mirror" {
          timing: w2479 -> [_]
          timing-out: [_] -> w2478
          tunnel: w2477 -> [w2480]
          i -> [w2518]
          stop <- w2481 stop-if-true
          n1663 = node-c288() -> (w2517:i64)  [unwired: 1 out]
          n1664 = Multiply(x="AO1", y=32767.0) -> (x*y=w2513:dbl)
          n1665 = Multiply(x="AO2", y=32767.0) -> (x*y=w2508:dbl)
          n1666 = Divide(x=w2513, y=10.0) -> (x/y=w2514:dbl)
          n1667 = Divide(x=w2508, y=10.0) -> (x/y=w2509:dbl)
          n1668 = To Word Integer(number=w2514) -> (16bit integer=w2506:i16)
          n1669 = To Word Integer(number=w2509) -> (16bit integer=w2505:i16)
          n1670 = Divide(x=w2517, y=i64 1000) -> (x/y=w2488:dbl)
          n1671 = Multiply(x=w2488, y=w2518) -> (x*y=w2499:dbl)
          n1672 = Multiply(x="Osc. freq. (Hz) 2", y=6.283185307179586) -> (x*y=w2500:dbl)
          n1673 = Multiply(x=w2500, y=w2499) -> (x*y=w2498:dbl)
          n1674 = Sine(x=w2498) -> (sin(x)=w2497:dbl)
          n1675 = Multiply(x=w2497, y="Osc. amp. (V)") -> (x*y=w2495:dbl)
          n1676 = Add(x=w2495, y="Osc. center (V)") -> (x+y=w2493:dbl)
          n1677 = Divide(x=w2493, y=10.0) -> (x/y=w2491:dbl)
          n1678 = Multiply(x=w2491, y=32767.0) -> (x*y=w2486:dbl)
          n1679 = Select(t=w2486, s="Scan axis", f=w2506) -> (s? t:f=w2504:dbl)
          n1680 = Select(t=w2505, s="Scan axis", f=w2486) -> (s? t:f=w2503:dbl)
          n1681 = local read "MCL Mode"() -> (w2485:u16)
          n1682 = Not Equal?(x=w2485, y=u16 1) -> (x != y?=w2482:bool)
          n1683 = local read "Stop All"() -> (w2483:bool)
          n1684 = xnode "Read/Write Control"("FPGA VI Reference In"=w2480, "AO1"=w2504, "AO2"=w2503) -> ()  [unwired: 1 in, 2 out]
          n1685 = Compound Arithmetic op=OR(w2483, w2482) -> (w2481:bool)
          n1686 = node-c288() -> ()  [unwired: 2 out]
        }
        n1687 = node-c288(w2478) -> ()  [unwired: 1 out]
      }
      frame 2 {
        n1688 = case shown="True" "Start Scan" {
          tunnel: w2524 -> [_ w2526]
          frame False {
          }
          frame True {
            n1689 = Subtract(x="End (V)", y="Begin (V)") -> (x-y=w2533:dbl)
            n1690 = Decrement(x="N Points") -> (x-1=w2532:dbl)
            n1691 = Divide(x=w2533, y=w2532) -> (x/y=w2530:dbl)
            n1692 = for {
              N: "N Points" -> [_]
              tunnel: "Begin (V)" -> [w2549]
              tunnel: [w2541] -> w2536 mode=indexing
              tunnel: w2530 -> [w2540]
              tunnel: [w2538] -> w2529 mode=indexing
              tunnel: w2526 -> [w2537]
              i -> [w2548]
              n1693 = Multiply(x=w2540, y=w2548) -> (x*y=w2547:dbl)
              n1694 = Add(x=w2549, y=w2547) -> (x+y=w2544:dbl)
              n1695 = local read "Scan axis"() -> (w2539:bool)
              n1696 = local read "AO1"() -> (w2546:dbl)
              n1697 = local read "AO2"() -> (w2545:dbl)
              n1698 = Select(t=w2544, s=w2539, f=w2546) -> (s? t:f=w2543:dbl)
              n1699 = Select(t=w2545, s=w2539, f=w2544) -> (s? t:f=w2542:dbl)
              n1700 = flat-sequence {
                tunnel: w2543 -> [w2553]
                tunnel: w2542 -> [w2552]
                tunnel: w2537 -> [w2550]
                tunnel: [w2563] -> w2541
                tunnel: [w2562] -> w2538
                frame #0 {
                  w2556 = 10.0 ("y")
                  w2551 = 32767.0 ("y")
                  n1701 = Multiply(x=w2553, y=w2551) -> (x*y=w2559:dbl)
                  n1702 = Multiply(x=w2552, y=w2551) -> (x*y=w2557:dbl)
                  n1703 = Divide(x=w2559, y=w2556) -> (x/y=w2560:dbl)
                  n1704 = Divide(x=w2557, y=w2556) -> (x/y=w2558:dbl)
                  n1705 = To Word Integer(number=w2560) -> (16bit integer=w2554:i16)
                  n1706 = To Word Integer(number=w2558) -> (16bit integer=w2555:i16)
                  n1707 = xnode "Read/Write Control"("FPGA VI Reference In"=w2550, "AO1"=w2554, "AO2"=w2555) -> ()  [unwired: 1 in, 2 out]
                }
                frame #1 {
                  n1708 = Wait (ms)(milliseconds to wait="DAQ Delay (ms)") -> ()  [unwired: 1 out]
                }
                frame #2 {
                  n1709 = local read "Slow mean"() -> (w2563:dbl)
                  n1710 = local read "Sigma"() -> (w2562:dbl)
                }
              }
            }
            n1711 = Bundle("Begin (V)"="Begin (V)", w2530, w2536) -> (→"MCL Scan":cluster{"Begin (V)":dbl, dbl, dbl[]})  [unwired: 1 out]
            n1712 = Bundle("Begin (V)"="Begin (V)", w2530, w2529) -> (→"MCL Scan 2":cluster{"Begin (V)":dbl, dbl, dbl[]})  [unwired: 1 out]
          }
        }
      }
    }
    n1713 = local read "Stop All"() -> (w2474:bool)
    n1714 = node-c288() -> ()  [unwired: 2 out]
  }
  n1715 = timed-loop "Mouse control: trap position (AOM deflection), set confocal spot from image" {
    tunnel: [w2565] -> w86
    timing: w80 -> [_]
    timing-out: [_] -> w79
    tunnel: w17 -> [w2564]
    stop <- w2565 stop-if-true
    n1716 = node-c288() -> ()  [unwired: 2 out]
    n1717 = event shown="[0] \"Pane\": Mouse Down" {
      selector: _ -> [_ _]
      dyn-events: _ -> [_ _]
      timeout: _ -> [_ _]
      tunnel: w2564 -> [w2568 _]
      event Mouse Down {
        n1718 = event-data() -> ("Time"=w2570:u32, "Coords"=w2569:T9, "Button"=w2571:u16)  [unwired: 6 out]
        n1719 = case shown="3" w2571 {
          tunnel: w2570 -> [_ _ w2677]
          tunnel: w2569 -> [_ w2608 w2675]
          tunnel: w2568 -> [_ _ w2671]
          frame 0, Default {
          }
          frame 1 {
            n1720 = property on="APD 2" class="ImageControl"() -> ("Displayed Image Position"=w2578:cluster{"Left":i32, "Top":i32})  [unwired: 2 in, 2 out]
            n1721 = property on="APD 1" class="ImageControl"() -> ("Displayed Image Position"=w2607:cluster{"Left":i32, "Top":i32})  [unwired: 2 in, 2 out]
            n1722 = property on="Detection Laser X" class="ImageControl"() -> ("Displayed Image Position"=w2604:cluster{"Left":i32, "Top":i32})  [unwired: 2 in, 2 out]
            n1723 = property on="Detection Laser Y" class="ImageControl"() -> ("Displayed Image Position"=w2603:cluster{"Left":i32, "Top":i32})  [unwired: 2 in, 2 out]
            n1724 = property on="APD 2" class="ImageControl"() -> ("Displayed Image Size"=w2577:cluster{"Width":u32, "Height":u32})  [unwired: 2 in, 2 out]
            n1725 = property on="APD 1" class="ImageControl"() -> ("Displayed Image Size"=w2605:cluster{"Width":u32, "Height":u32})  [unwired: 2 in, 2 out]
            n1726 = property on="Detection Laser X" class="ImageControl"() -> ("Displayed Image Size"=w2606:cluster{"Width":u32, "Height":u32})  [unwired: 2 in, 2 out]
            n1727 = property on="Detection Laser Y" class="ImageControl"() -> ("Displayed Image Size"=w2602:cluster{"Width":u32, "Height":u32})  [unwired: 2 in, 2 out]
            n1728 = Unbundle By Name(w2577) -> ("Width"=w2574:u32, "Height"=w2573:u32)
            n1729 = Unbundle By Name(w2578) -> ("Left"=w2576:i32, "Top"=w2575:i32)
            n1730 = Unbundle By Name(w2605) -> ("Width"=w2599:u32, "Height"=w2598:u32)
            n1731 = Unbundle By Name(w2606) -> ("Width"=w2595:u32, "Height"=w2594:u32)
            n1732 = Unbundle By Name(w2602) -> ("Width"=w2591:u32, "Height"=w2590:u32)
            n1733 = Unbundle By Name(w2607) -> ("Left"=w2601:i32, "Top"=w2600:i32)
            n1734 = Unbundle By Name(w2604) -> ("Left"=w2597:i32, "Top"=w2596:i32)
            n1735 = Unbundle By Name(w2603) -> ("Left"=w2593:i32, "Top"=w2592:i32)
            n1736 = Bundle("Left"=w2576, "Top"=w2575, "Width"=w2574, "Height"=w2573) -> (w2572:T37)  [unwired: 1 in]
            n1737 = Bundle("Left"=w2601, "Top"=w2600, "Width"=w2599, "Height"=w2598) -> (w2589:T37)  [unwired: 1 in]
            n1738 = Bundle("Left"=w2597, "Top"=w2596, "Width"=w2595, "Height"=w2594) -> (w2588:T37)  [unwired: 1 in]
            n1739 = Bundle("Left"=w2593, "Top"=w2592, "Width"=w2591, "Height"=w2590) -> (w2587:T37)  [unwired: 1 in]
            n1740 = Build Cluster Array(w2572, w2589, w2588, w2587) -> (w2586:T38)
            n1741 = for {
              tunnel: w2608 -> [w2619]
              tunnel: w2586 -> [w2620] mode=indexing
              shift-right: [w2617] -> w2584
              shift-left: TRUE -> [w2618]
              shift-right: [w2616] -> w2582
              shift-left: _ -> [w2612]
              shift-right: [w2615] -> w2581
              shift-left: _ -> [w2611]
              shift-right: [w2614] -> w2580
              shift-left: _ -> [w2610]
              shift-right: [w2613] -> w2579
              shift-left: _ -> [w2609]
              n1742 = case shown="True" w2618 {
                selector: w2618 -> [w2625 _]
                tunnel: w2620 -> [_ w2634]
                tunnel: w2619 -> [_ w2632]
                tunnel: [w2625 w2630] -> w2617
                tunnel: [w2624 w2629] -> w2616
                tunnel: [w2623 w2628] -> w2615
                tunnel: [w2622 w2627] -> w2614
                tunnel: [w2621 w2626] -> w2613
                tunnel: w2612 -> [w2624 _]
                tunnel: w2611 -> [w2623 _]
                tunnel: w2610 -> [w2622 _]
                tunnel: w2609 -> [w2621 _]
                frame False {
                }
                frame True {
                  n1743 = Unbundle(w2634) -> (w2633:T37)
                  n1744 = call "isclickinwindow.vi"("Image Param"=w2633, "Point32"=w2632) -> ("4 Y"=w2626:i32, "3 Height"=w2627:i32, "2 X"=w2628:i32, "1 Width"=w2629:i32, "In image?"=w2631:bool)  [unwired: 1 in]
                  n1745 = Not(x=w2631) -> (.not. x?=w2630:bool)
                }
              }
            }
            n1746 = Not(x=w2584) -> (.not. x?=w2583:bool)
            n1747 = case shown="True" w2583 {
              tunnel: w2581 -> [_ w2648]
              tunnel: w2579 -> [_ w2647]
              tunnel: w2582 -> [_ w2646]
              tunnel: w2580 -> [_ w2645]
              frame False {
              }
              frame True {
                w2635 = FALSE ("Get Point")
                n1748 = local read "Scan lines (y)"() -> (w2650:u64)
                n1749 = disable-structure shown="Disabled" {